vi "Joystick and Camera.vi"(6 "XYZTheta":dbl[](array[numeric])) -> (1 "Gantry":dbl[](array[numeric])=[1219.240705557797, 722.8421823618999, 52.864847366341415, 0.003106741190800654] format="%#_8g", 2 "Sum":dbl[](array[numeric])=[1219.30639899585, 722.8896830877354, 52.864847366341415, 0.003106741190800654] format="%#_8g")   [LabVIEW 2016]
uses:
  Classes/Controller/Camera/Camera Folder/Machine Vision.ctl
  <vilib>/Utility/file.llb/Write Delimited Spreadsheet (DBL).vi
  Classes/Controller/I-O/I-O Folder/I-O.lvclass
  Classes/Controller/Motion/Motion Folder/Motion.lvclass
  Classes/Controller/Camera/Camera Folder/Camera.lvclass
  Classes/Controller/Controller Folder/Controller.lvclass
panel:
  in  "input":dbl
  in  "Camera light":bool
  in  "Go 3":bool
  in  "file path (dialog if empty) 3":path
  out "Bellow offset":dbl[](array[numeric])
  out "Camera 2":dbl[](array[numeric])=[0.0, 0.0, 52.864847366341415, 0.003106741190800654] format="%#_8g"
  out "Camera 1":dbl[](array[numeric])=[0.0, 0.0, 52.864847366341415, 0.003106741190800654] format="%#_8g"
  out "Bellow position":dbl[](array[numeric])=[0.0, 0.0, 52.864847366341415, 0.003106741190800654] format="%#_8g"
  in  "Record 2":bool
  in  "Record 1":bool
  in  "Pickup & Rotate":bool
  in  "Write to file":bool
  out "XYZTheta Out":dbl[](array[numeric])
  out "Waveform Graph":dbl[](graph)
  out "Array 2":dbl[](array[numeric])
  out "Array":dbl[](array[numeric])
  out "Numeric":dbl
  out "Image 2":T1(plugin-control)
  in  "Machine Vision 2":T2=enum."tpcb_hole"
  in  "interval":dbl
  in  "focus":bool
  in  "On/Off":bool=TRUE
  in  "Vacuum":bool
  out "Record Times":i32
  in  "Channel":i32=20
  in  "Filename":path=path "test.lvm"
  in  "Record":bool
  in  "Go 2":bool
  in  "Z Go":bool
  in  "Position":dbl
  in  "Machine Vision":T2=enum."tpcb_hole"
  in  "Go":bool
  in  "Joystick":bool
  in  "Stop":bool
  out "Image":T1(plugin-control)
  out "Camera":dbl[](array[numeric])=[0.23163148760795593, 0.18427667021751404] format="%#_8g"
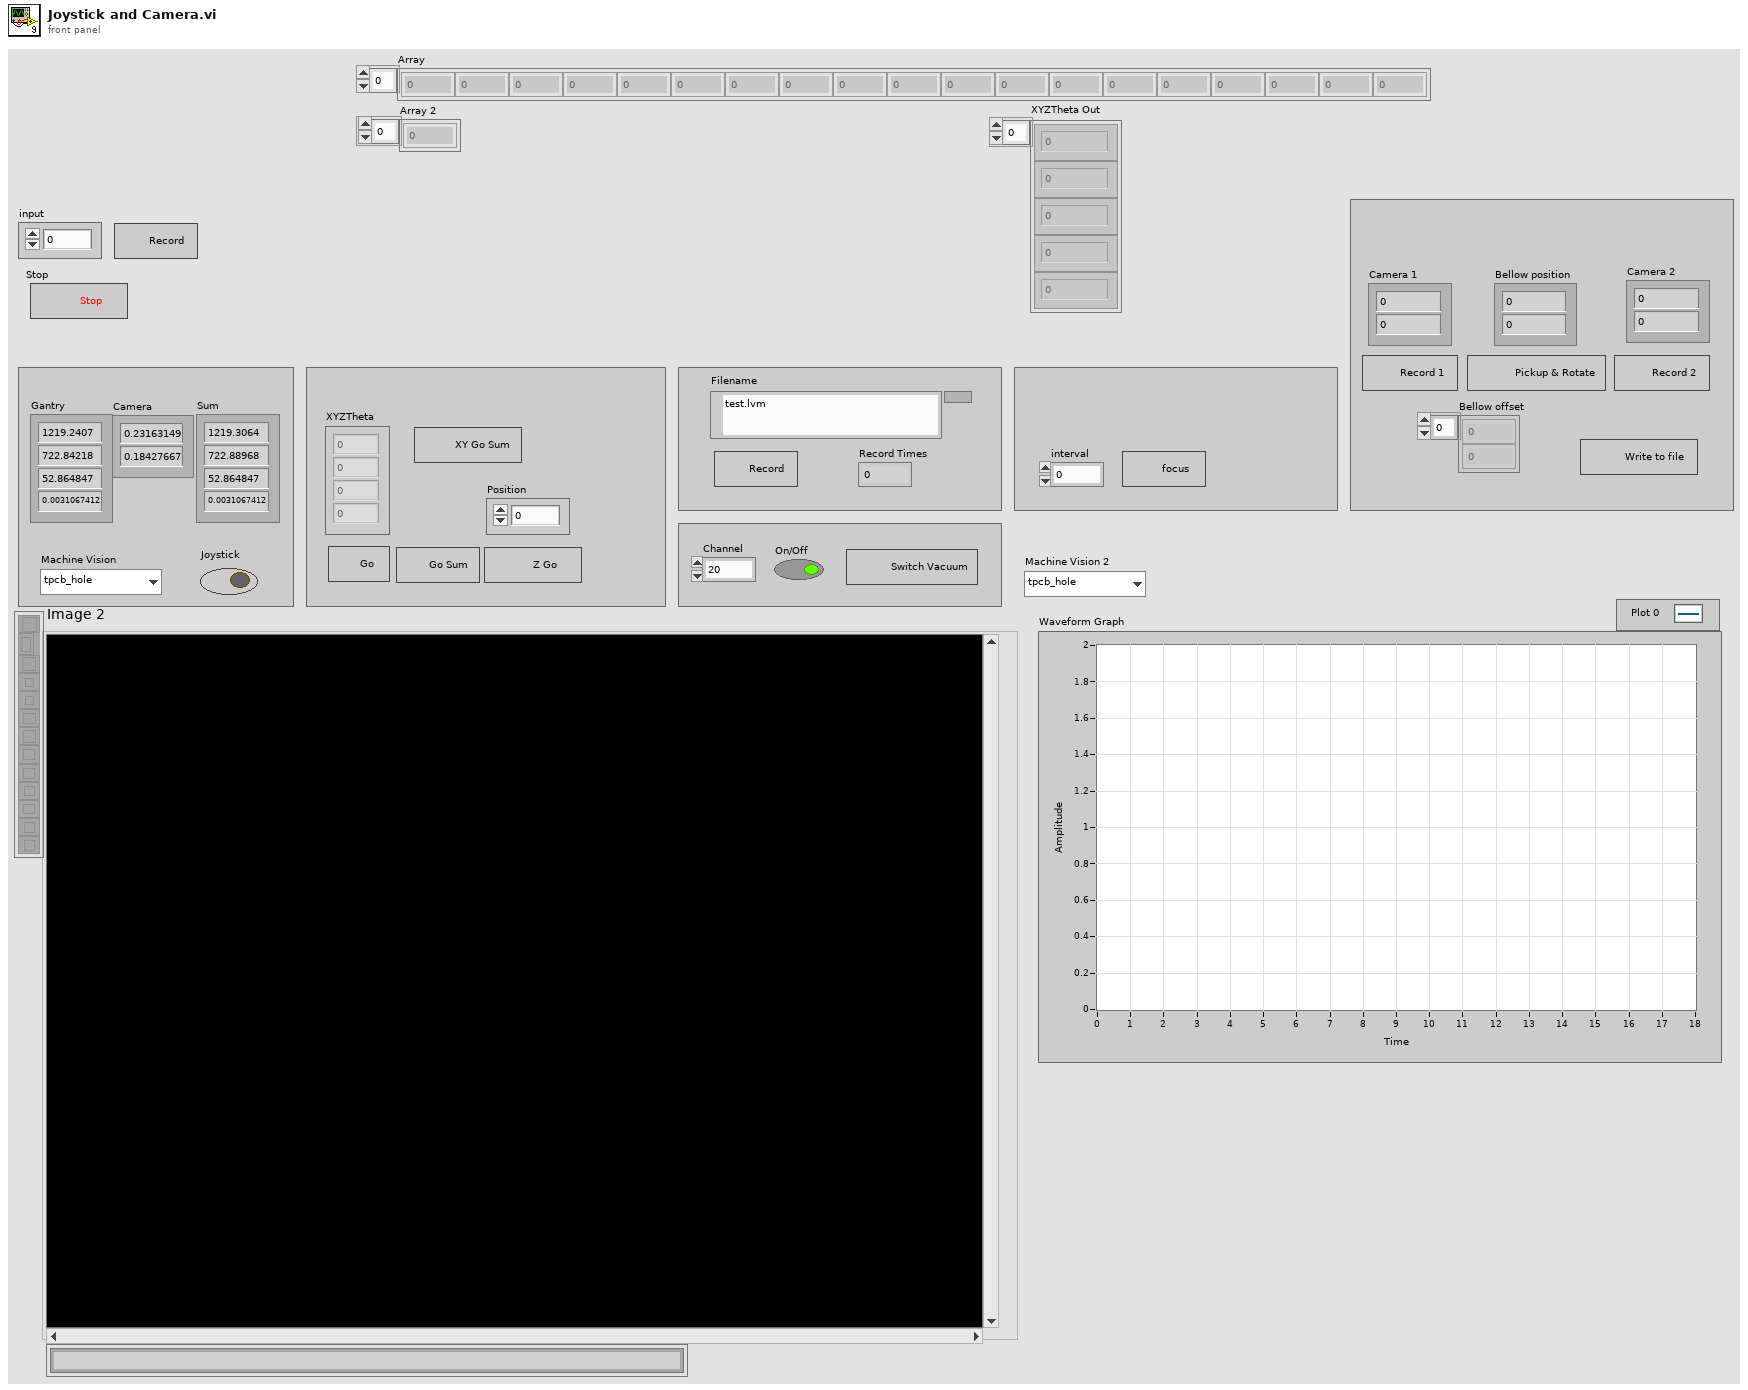
[diagram p1: front panel]
types:
  T1 = typedef "IMAQ Image.ctl" = refnum<image>
  T2 = typedef "Camera.lvclass/Machine Vision.ctl" = enum16{"top left corner", "top right corner", "bottom left corner", "bottom right corner", "bottom left chip", "top right chip", "None", "tracker fiducial", "chip cross 2", "chip cross", "Focus", "INTT HDI Mark", "INTT Sensor Cross", "INTT Chip Corner", "HPK Silicon", "Circle", "tpcb_hole"}
  T3 = typedef "Controller.lvclass/Controllers.ctl" = cluster{"Copy of Motion.lvclass":refnum<class "Motion.lvclass">, "Copy of I-O.lvclass ":refnum<class "I-O.lvclass">, "Copy of Dispenser.lvclass":refnum<class "Dispenser.lvclass">}
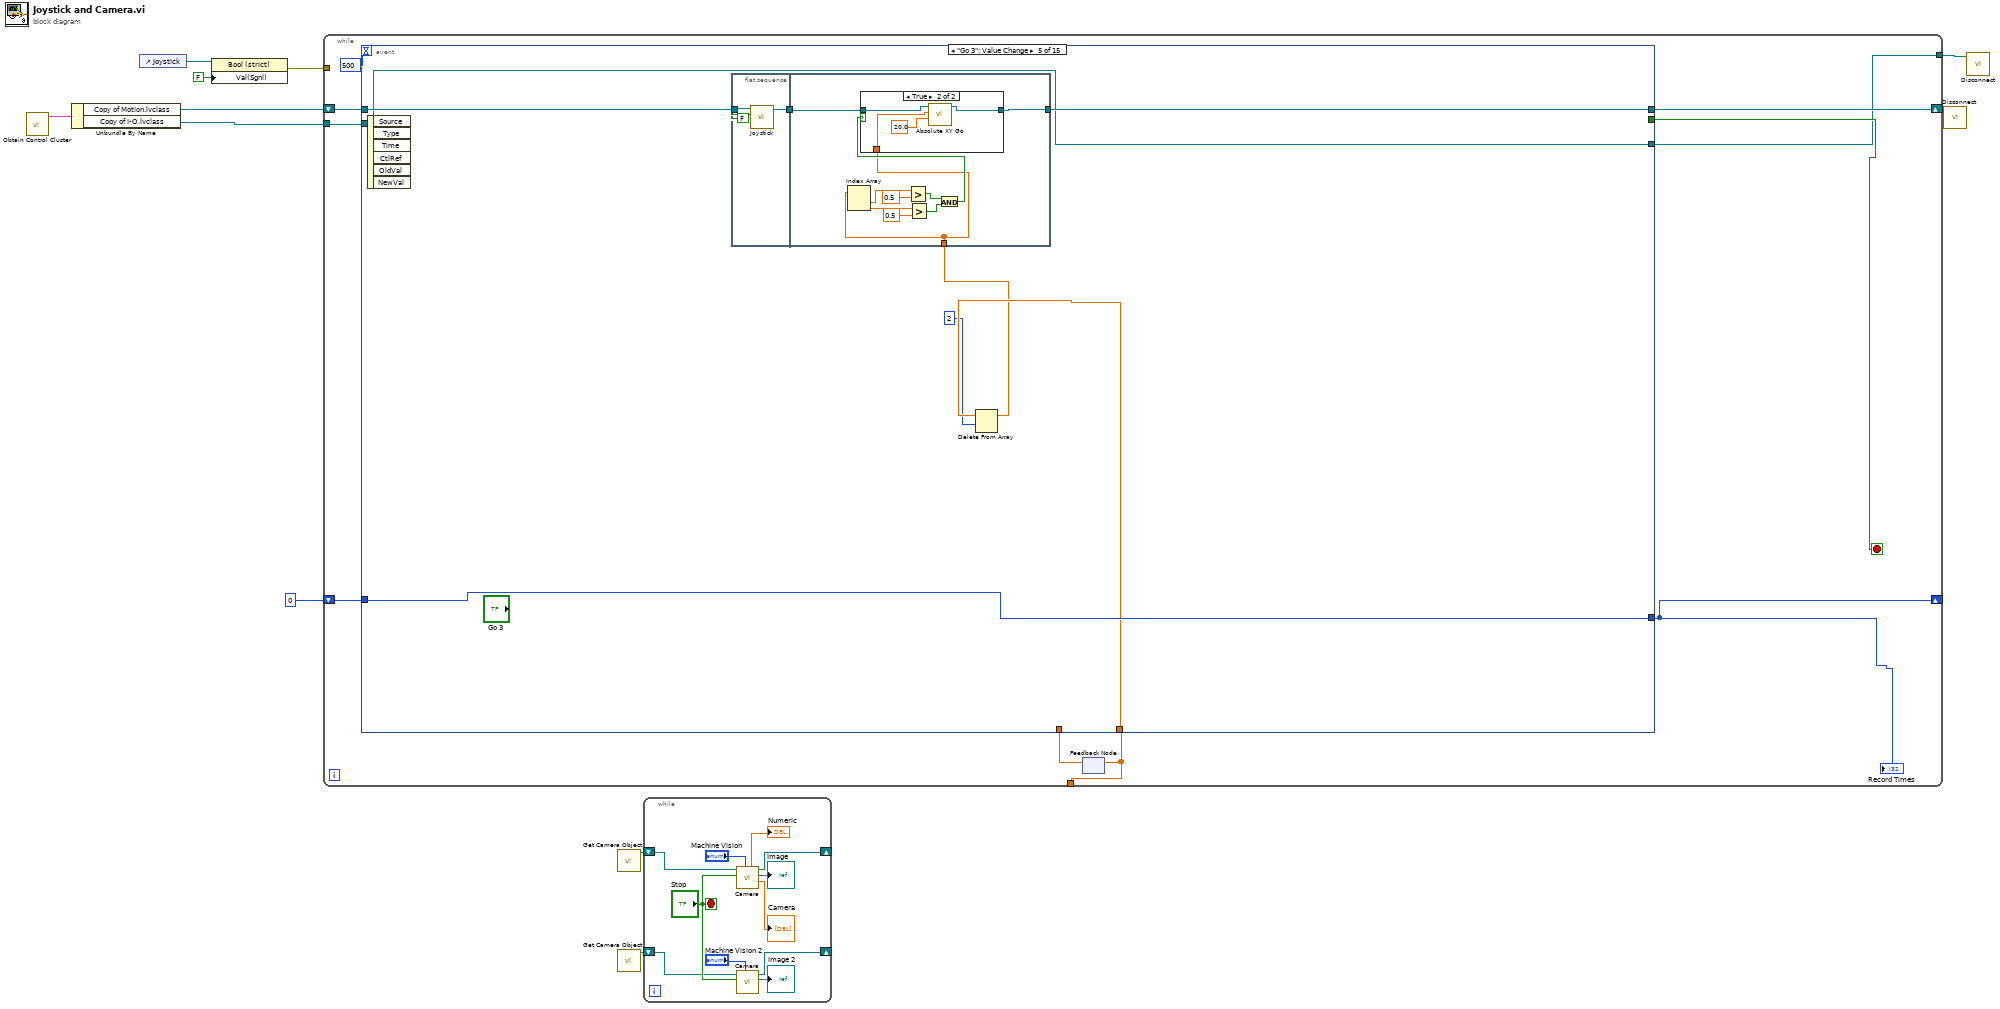
[diagram p0: block diagram]
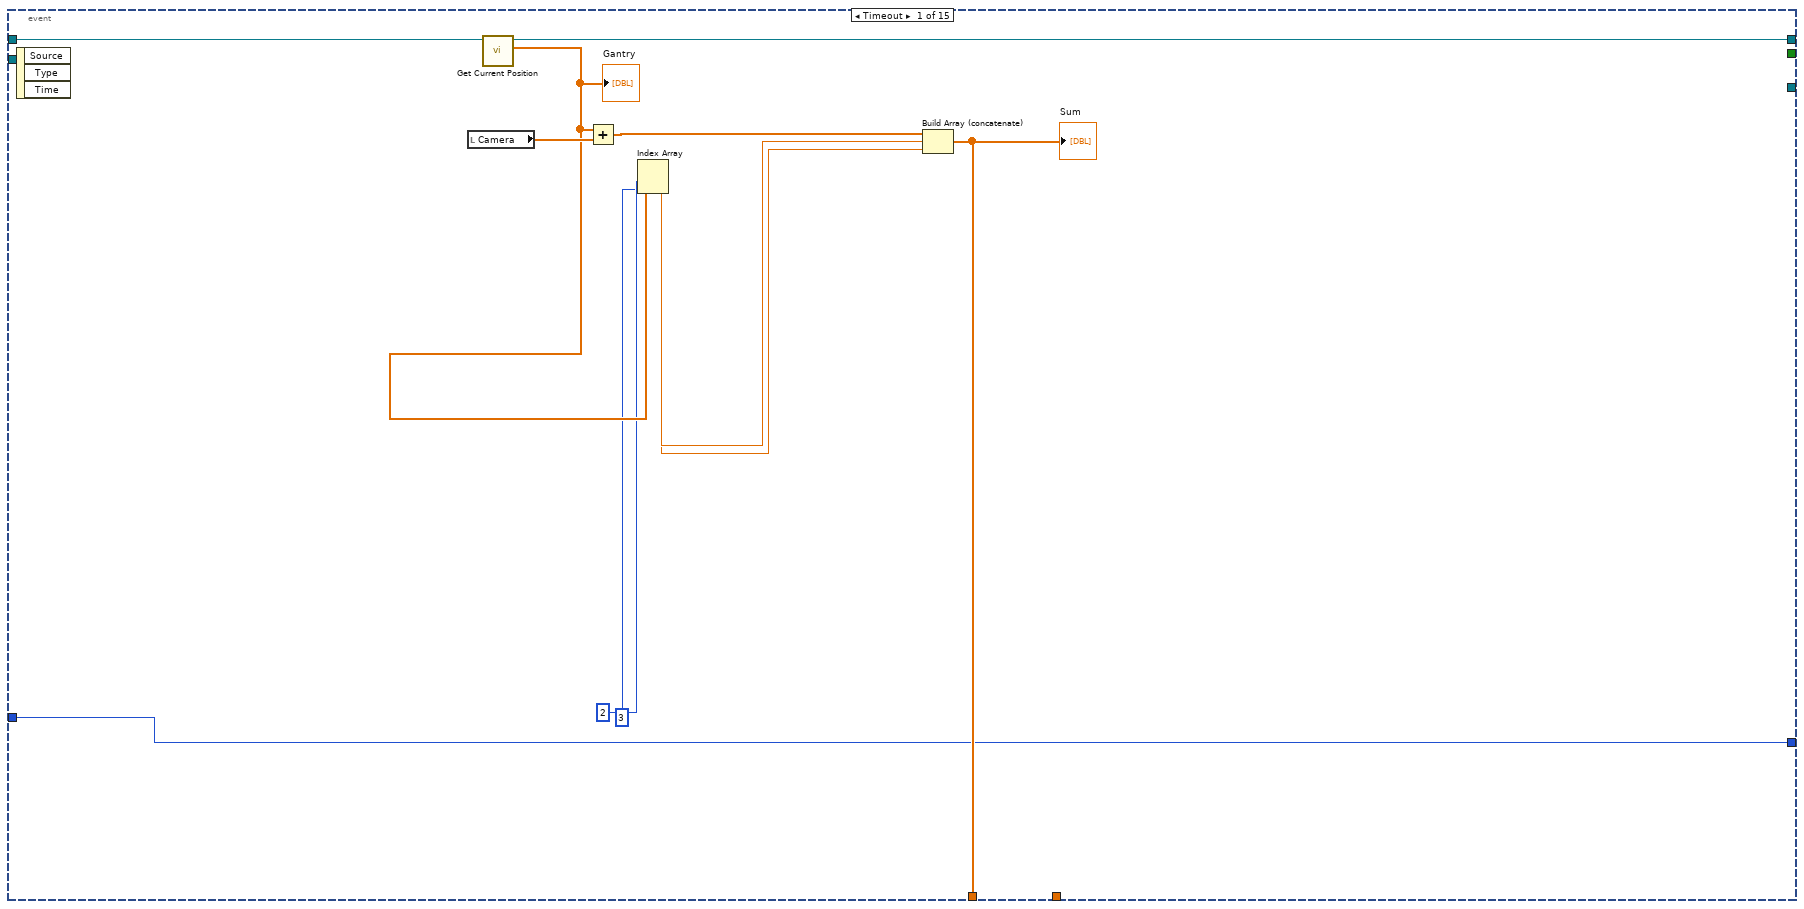
[diagram p2: hidden frame]
diagram:
  n1 = call "Obtain Control Cluster.vi"() -> ("Control Out"=w7:T3)  [unwired: 11 in]
  n2 = Unbundle By Name(w7) -> ("Copy of Motion.lvclass"=w6:refnum<class "Motion.lvclass">, "Copy of I-O.lvclass"=w2:refnum<class "I-O.lvclass">)
  n3 = control-ref of="Joystick"() -> (w10:refnum<vi>)
  n4 = property class="Bool (strict)"(reference=w10, "Val(Sgnl)"=FALSE ("Value (Signaling)")) -> (error out=w9:errorcluster)  [unwired: 1 in, 1 out]
  n5 = while {
    shift-right: [w19] -> w5
    shift-left: w6 -> [w16]
    tunnel: w9 -> [_]
    tunnel: [w18] -> _
    tunnel: w2 -> [w13]
    shift-right: [w14] -> _
    shift-left: 0 -> [w15]
    tunnel: [w12] -> w3
    stop <- w20 stop-if-true
    n6 = feedback #1() -> (w18:dbl[])  [unwired: 1 in]
    n7 = event shown="[4] \"Go 3\": Value Change" {
      selector: _ -> [_ _ _ _ _ _ _ _ _ _ _ _ _ _ _]
      dyn-events: _ -> [_ _ _ _ _ _ _ _ _ _ _ _ _ _ _]
      timeout: 500 -> [_ _ _ _ _ _ _ _ _ _ _ _ _ _ _]
      tunnel: [_ _ _ _ _ _ _ _ _ _ _ _ _ _ TRUE] -> w20
      tunnel: w16 -> [w31 w37 w42 w64 w78 w101 w105 w111 w162 w168 w172 w185 w210 w226 w229]
      tunnel: [w30 w35 w41 w63 w77 w100 w105 w119 w162 w168 w172 w185 w199 w226 w227] -> w19
      tunnel: [w26 _ _ _ _ _ _ _ _ _ _ _ _ _ _] -> w17
      tunnel: w18 -> [_ _ _ w61 w74 _ w107 _ _ _ _ _ _ _ _]
      tunnel: w15 -> [w22 w34 w39 w60 w75 w97 w103 _ _ _ _ _ _ w224 _]
      tunnel: [w22 w34 w39 w60 w75 w97 w102 _ _ _ _ _ _ w224 _] -> w14
      tunnel: w13 -> [_ w33 w38 w59 w71 _ _ _ w166 w167 w171 w184 w208 w225 _]
      tunnel: [_ w33 w38 w59 w71 _ _ _ w165 w167 w171 w184 w192 w225 _] -> w12
      event Timeout {
        n8 = event-data() -> ()  [unwired: 1 in, 3 out]
        n9 = local read "Camera"() -> (w32:dbl[])
        n10 = call-dynamic "Get Current Position.vi"("Motion in"=w31) -> ("XYZTheta Out"=w28:dbl[], "Motion out"=w30:refnum<class "Motion.lvclass">)  [unwired: 8 in, 1 out]
        "Gantry" <- w28
        n11 = Add(x=w28, y=w32) -> (x+y=w29:dbl[])
        n12 = Index Array(array=w28, index #1=2 ("index"), index #2=3 ("index")) -> (element #1=w24:dbl, element #2=w23:dbl)
        n13 = Build Array (concatenate)(w29, w24, w23) -> (w26:dbl[])
        "Sum" <- w26
      }
      event "Joystick": Value Change {
        n14 = event-data() -> ()  [unwired: 1 in, 6 out]
        n15 = call-dynamic "Joystick.vi"("Joystick"="Joystick", "Motion in"=w37) -> ("Motion out"=w35:refnum<class "Motion.lvclass">)  [unwired: 8 in, 1 out]
      }
      event "Go": Value Change {
        n16 = event-data() -> ()  [unwired: 1 in, 6 out]
        n17 = flat-sequence {
          tunnel: w42 -> [w44]
          tunnel: [w43] -> w40
          tunnel: [w46] -> w41
          tunnel: w40 -> [w49]
          frame #0 {
            n18 = call-dynamic "Joystick.vi"("Joystick"=FALSE, "Motion in"=w44) -> ("Motion out"=w43:refnum<class "Motion.lvclass">)  [unwired: 8 in, 1 out]
          }
          frame #1 {
            n19 = for {
              tunnel: "XYZTheta" -> [w56] mode=indexing
              tunnel: [w54] -> w48 mode=indexing
              shift-right: [w52] -> w47
              shift-left: w49 -> [w53]
              i -> [w58]
              n20 = Equal To 0?(x=w56) -> (x = 0?=w57:bool)
              n21 = call-dynamic "Get Current Position.vi"("Motion in"=w53) -> ("XYZTheta Out"=w51:dbl[], "Motion out"=w52:refnum<class "Motion.lvclass">)  [unwired: 8 in, 1 out]
              n22 = Index Array(array=w51, index=w58) -> (element=w55:dbl)
              n23 = Select(t=w55, s=w57, f=w56) -> (s? t:f=w54:dbl)
            }
            n24 = call "XYZTheta Go.vi"("XYZTheta In"=w48, "Motion in"=w47) -> ("Motion out"=w46:refnum<class "Motion.lvclass">)  [unwired: 7 in, 2 out]
          }
        }
      }
      event "Go 2": Value Change {
        n25 = event-data() -> ()  [unwired: 1 in, 6 out]
        n26 = flat-sequence {
          tunnel: w64 -> [w66]
          tunnel: [w65] -> w62
          tunnel: [w70] -> w63
          tunnel: w62 -> [w69]
          tunnel: w61 -> [w68]
          frame #0 {
            n27 = call-dynamic "Joystick.vi"("Joystick"=FALSE, "Motion in"=w66) -> ("Motion out"=w65:refnum<class "Motion.lvclass">)  [unwired: 8 in, 1 out]
          }
          frame #1 {
            n28 = call "XYZTheta Go.vi"("XYZTheta In"=w68, "Motion in"=w69) -> ("Motion out"=w70:refnum<class "Motion.lvclass">)  [unwired: 7 in, 2 out]
          }
        }
      }
      event "Go 3": Value Change {
        n29 = event-data() -> ()  [unwired: 1 in, 6 out]
        n30 = flat-sequence {
          tunnel: w78 -> [w80]
          tunnel: [w79] -> w76
          tunnel: [w90] -> w77
          tunnel: w76 -> [w91]
          tunnel: w72 -> [w82]
          frame #0 {
            n31 = call-dynamic "Joystick.vi"("Joystick"=FALSE, "Motion in"=w80) -> ("Motion out"=w79:refnum<class "Motion.lvclass">)  [unwired: 8 in, 1 out]
          }
          frame #1 {
            n32 = Index Array(array=w82) -> (element #1=w89:dbl, element #2=w87:dbl)  [unwired: 2 in]
            n33 = Greater?(x=w89, y=0.5) -> (0:w85:bool)
            n34 = Greater?(x=w87, y=0.5) -> (0:w84:bool)
            n35 = And(x=w85, y=w84) -> (x .and. y?=w83:bool)
            n36 = case shown="True" w83 {
              tunnel: w91 -> [w92 w96]
              tunnel: [w92 w95] -> w90
              tunnel: w82 -> [_ w93]
              frame False {
              }
              frame True {
                n37 = call-dynamic "Absolute XY Go.vi"("Speed"=20.0, "XY"=w93, "Motion in"=w96) -> ("Motion out"=w95:refnum<class "Motion.lvclass">)  [unwired: 7 in, 1 out]
              }
            }
          }
        }
        n38 = Delete From Array(array=w74, length=2) -> (array with subset deleted=w72:dbl[])  [unwired: 1 in, 1 out]
      }
      event "Z Go": Value Change {
        n39 = event-data() -> ()  [unwired: 1 in, 6 out]
        n40 = call-dynamic "Z Go.vi"("Speed"=2.0, "Position"="Position", "Motion in"=w101) -> ("Motion out"=w100:refnum<class "Motion.lvclass">)  [unwired: 7 in, 1 out]
      }
      event "Record": Value Change {
        n41 = event-data() -> ()  [unwired: 1 in, 6 out]
        n42 = Increment(x=w103) -> (x+1=w102:i32)
        n43 = call-poly <vilib>:"Write Delimited Spreadsheet.vi"("file path (dialog if empty)"="Filename", "format (%.3f)"="%.4f", "1D data"=w107, "append to file? (new file:F)"=TRUE) -> ()  [unwired: 10 in, 2 out]
      }
      event "focus": Value Change {
        (unwired) FALSE ("Joystick")
        n44 = event-data() -> ()  [unwired: 1 in, 6 out]
        n45 = call-dynamic "Joystick.vi"("Motion in"=w111) -> ("Motion out"=w110:refnum<class "Motion.lvclass">)  [unwired: 9 in, 1 out]
        n46 = Multiply(x="interval", y=-10) -> (x*y=w127:dbl)
        n47 = Build Array(w127) -> (w129:dbl[])
        n48 = call-dynamic "wrtCurrent Go.vi"("Axis"=string[] ["Z"], "Speed"=10.0, "Distance"=w129, "Motion in"=w110) -> ("Motion out"=w133:refnum<class "Motion.lvclass">)  [unwired: 6 in, 1 out]
        n49 = for {
          N: 19 -> [_]
          tunnel: w133 -> [w136]
          tunnel: [w140] -> w118
          shift-right: [w137] -> w125
          shift-left: dbl[] [] -> [w138]
          tunnel: "interval" -> [w143]
          tunnel: [w139] -> _
          n50 = for {
            N: 7 -> [_]
            shift-right: [w157] -> w148
            shift-left: dbl[] [] -> [w156]
            n51 = flat-sequence {
              tunnel: w156 -> [w159]
              tunnel: [w160] -> w155
              tunnel: [w161] -> w157
              tunnel: w155 -> [w161]
              frame #0 {
                n52 = local read "Numeric"() -> (w158:dbl)
                n53 = Insert Into Array(array=w159, new element=w158) -> (w160:dbl[])  [unwired: 1 in]
              }
              frame #1 {
                n54 = call "Time Delay2"() -> ()  [unwired: 11 in, 1 out]
              }
            }
          }
          n55 = call-dynamic "Get Current Position.vi"("Motion in"=w136) -> ("XYZTheta Out"=→"XYZTheta Out":dbl[])  [unwired: 8 in, 2 out]
          n56 = Build Array(w143) -> (w142:dbl[])
          n57 = call-dynamic "wrtCurrent Go.vi"("Axis"=string[] ["Z"], "Speed"=10.0, "Distance"=w142, "Motion in"=w136) -> ("error out"=w149:errorcluster, "Motion out"=w140:refnum<class "Motion.lvclass">)  [unwired: 6 in]
          n58 = call "Convert to Dynamic Data"("Array"=w148) -> ("Dynamic Data Type"=w147:dynamicdata)  [unwired: 3 in]
          n59 = call "Statistics"("Signals"=w147) -> ("Arithmetic Mean"=w145:dynamicdata)  [unwired: 25 in, 1 out]
          n60 = call "Time Delay"("error in (no error)"=w149) -> ("error out"=w139:errorcluster)  [unwired: 10 in]
          n61 = call "Convert from Dynamic Data"("Dynamic Data Type"=w145) -> ("Array"=w141:dbl[])  [unwired: 3 in]
          n62 = for {
            tunnel: w141 -> [w154] mode=indexing
            shift-right: [w153] -> w137
            shift-left: w138 -> [w152]
            n63 = Insert Into Array(array=w152, new element=w154) -> (w153:dbl[])  [unwired: 1 in]
          }
          "Array" <- w137
          "Waveform Graph" <- w137
        }
        n64 = call "Convert to Dynamic Data2"("Array"=w125) -> ("Dynamic Data Type"=w124:dynamicdata)  [unwired: 3 in]
        n65 = call "Statistics2"("Signals"=w124) -> ("Index of Max"=w123:dynamicdata)  [unwired: 25 in, 1 out]
        n66 = call "Convert from Dynamic Data2"("Dynamic Data Type"=w123) -> ("Array"=w109:dbl[])  [unwired: 3 in]
        "Array 2" <- w109
        n67 = Index Array(array=w109, index=0) -> (element=w113:dbl)
        n68 = local read "interval"() -> (w116:dbl)
        n69 = Subtract(x=w113, y=18.0 ("x")) -> (x-y=w117:dbl)
        n70 = Multiply(x=w116, y=w117) -> (x*y=w115:dbl)
        n71 = Build Array(w115) -> (w114:dbl[])
        n72 = call-dynamic "wrtCurrent Go.vi"("Axis"=string[] ["Z"], "Speed"=10.0, "Distance"=w114, "Motion in"=w118) -> ("Motion out"=w119:refnum<class "Motion.lvclass">)  [unwired: 6 in, 1 out]
      }
      event "Vacuum": Value Change {
        n73 = event-data() -> ()  [unwired: 1 in, 6 out]
        n74 = call-dynamic "Digital Write 1 Channel.vi"("Value"="On/Off", "Channel"="Channel", "I-O.lvclass"=w166) -> ("I-O.lvclass 2"=w165:refnum<class "I-O.lvclass">)  [unwired: 7 in, 1 out]
      }
      event "Record 1": Value Change {
        n75 = event-data() -> ()  [unwired: 1 in, 6 out]
        n76 = local read "Gantry"() -> (→"Bellow position":dbl[])
        n77 = local read "Sum"() -> (→"Camera 1":dbl[])
      }
      event "Record 2": Value Change {
        n78 = event-data() -> ()  [unwired: 1 in, 6 out]
        n79 = local read "Sum"() -> (→"Camera 2":dbl[])
      }
      event "Write to file": Value Change {
        n80 = event-data() -> ()  [unwired: 1 in, 6 out]
        n81 = local read "Camera 1"() -> (w188:dbl[])
        n82 = local read "Camera 2"() -> (w187:dbl[])
        n83 = local read "Bellow position"() -> (w182:dbl[])
        n84 = Add(x=w188, y=w187) -> (x+y=w186:dbl[])
        n85 = Divide(x=w186, y=2.0) -> (x/y=w183:dbl[])
        n86 = Subtract(x=w182, y=w183) -> (x-y=w181:dbl[])
        n87 = Index Array(array=w181, index #1=0 ("index"), index #2=1 ("index")) -> (element #1=w178:dbl, element #2=w177:dbl)
        n88 = Build Array(w178, w177, 0.0 ("element"), 0.0 ("element")) -> (w174:dbl[])
        "Bellow offset" <- w174
        n89 = call-poly <vilib>:"Write Delimited Spreadsheet.vi"("file path (dialog if empty)"="file path (dialog if empty) 3", "1D data"=w174, "append to file? (new file:F)"=FALSE) -> ()  [unwired: 11 in, 2 out]
      }
      event "Pickup & Rotate": Value Change {
        n90 = event-data() -> ()  [unwired: 1 in, 6 out]
        n91 = call-dynamic "Joystick.vi"("Joystick"=FALSE, "Motion in"=w210) -> ("Motion out"=w209:refnum<class "Motion.lvclass">)  [unwired: 8 in, 1 out]
        n92 = call "Lower_Stop.vi"("I-O in"=w208, "Motion in"=w209) -> ("I-O out"=w207:refnum<class "I-O.lvclass">, "Motion out"=w206:refnum<class "Motion.lvclass">)  [unwired: 7 in, 1 out]
        n93 = call "WriteReadWait.vi"("Read Value"=TRUE, "Write Value"=TRUE, "Read"=1, "Write"=1, "I-O in"=w207) -> ("error out"=w217:errorcluster, "I-O out"=w205:refnum<class "I-O.lvclass">)  [unwired: 5 in]
        n94 = call-dynamic "wrtCurrent Go.vi"("Axis"=string[] ["Z"], "error in (no error)"=w217, "Speed"=10.0, "Distance"=dbl[] [-20.0], "Motion in"=w206) -> ("Motion out"=w214:refnum<class "Motion.lvclass">)  [unwired: 5 in, 1 out]
        n95 = call-dynamic "wrtCurrent Go.vi"("Axis"=string[] ["U"], "Speed"=10.0, "Distance"=dbl[] [180.0], "Motion in"=w214) -> ("Motion out"=w204:refnum<class "Motion.lvclass">)  [unwired: 6 in, 1 out]
        n96 = call "Lower_Stop.vi"("I-O in"=w205, "Motion in"=w204) -> ("I-O out"=w193:refnum<class "I-O.lvclass">, "Motion out"=w200:refnum<class "Motion.lvclass">)  [unwired: 7 in, 1 out]
        n97 = call-dynamic "wrtCurrent Go.vi"("Axis"=string[] ["Z"], "Speed"=10.0, "Distance"=dbl[] [-20.0], "Motion in"=w200) -> ("Motion out"=w199:refnum<class "Motion.lvclass">)  [unwired: 6 in, 1 out]
        n98 = call "WriteReadWait.vi"("Read Value"=FALSE, "Write Value"=FALSE, "Read"=1, "Write"=1, "I-O in"=w193) -> ("I-O out"=w192:refnum<class "I-O.lvclass">)  [unwired: 5 in, 1 out]
      }
      event "Camera light": Value Change {
        n99 = event-data() -> ()  [unwired: 1 in, 6 out]
        n100 = call "Camera Light.vi"("input"="input") -> ()  [unwired: 2 in, 1 out]
      }
      event "Stop": Value Change {
        n101 = event-data() -> ()  [unwired: 1 in, 5 out]
        n102 = call-dynamic "Joystick.vi"("Joystick"=FALSE, "Motion in"=w229) -> ("Motion out"=w227:refnum<class "Motion.lvclass">)  [unwired: 8 in, 1 out]
      }
    }
    "Record Times" <- w14
    n103 = feedback-in #1(w17) -> ()
  }
  n104 = call "Get Camera Object.vi"() -> ("Camera out"=w8:refnum<class "Camera.lvclass">)  [unwired: 10 in, 1 out]
  n105 = call "Get Camera Object.vi"() -> ("Camera out"=w1:refnum<class "Camera.lvclass">)  [unwired: 10 in, 1 out]
  n106 = while {
    shift-right: [w240] -> _
    shift-left: w8 -> [w241]
    shift-right: [w233] -> _
    shift-left: w1 -> [w234]
    stop <- "Stop" stop-if-true
    n107 = call "Camera.vi"("Machine Vision"="Machine Vision", "Stop"="Stop", "Camera in"=w241) -> ("Camera"=→"Camera":dbl[], "Image"=→"Image":T1, "Camera out"=w240:refnum<class "Camera.lvclass">, "Focus output"=→"Numeric":dbl)  [unwired: 4 in, 1 out]
    n108 = call "Camera.vi"("Machine Vision"="Machine Vision 2", "Stop"="Stop", "Camera in"=w234) -> ("Image"=→"Image 2":T1, "Camera out"=w233:refnum<class "Camera.lvclass">)  [unwired: 4 in, 3 out]
  }
  n109 = call-dynamic "Disconnect.vi"("Motion in"=w5) -> ()  [unwired: 9 in, 1 out]
  n110 = call-dynamic "Disconnect.vi"("I-O in"=w3) -> ()  [unwired: 9 in, 1 out]